vi "saved waveform analysis220915.vi"() -> ()   [LabVIEW 2024] (continued)
15774.841666666667, 15775.016666666666, 15774.108333333334, 15775.741666666667, 15777.991666666667, 15775.008333333333, 15781.708333333334, 15773.5, 15775.016666666666, 15770.058333333332, 15774.858333333334, 15789.625, 15781.283333333333, 15781.708333333334, 15784.266666666666, 15777.816666666668, 15776.033333333333, 15770.666666666666, 15776.8, 15864.675, 15911.983333333334, 15907.916666666666, 15908.383333333333, 15907.2, 15907.5, 15909.125, 15909.733333333334, 15911.133333333333, 15906.575, 15906.758333333333, 15910.95, 15902.566666666668, 15911.083333333334, 15905.275, 15902.716666666667, 15905.525, 15907.641666666666, 15912.85, 15907.9, 15907.341666666667, 15903.591666666667, 15905.575, 15913.883333333333, 15908.85, 15910.908333333333, 15908.683333333332, 15913.641666666666, 15901.641666666666, 15904.675, 15912.433333333332, 15909.3, 15912.441666666668, 15917.483333333334, 15911.675, 15913.625, 15908.708333333334, 15916.45, 15909.591666666667, 15907.508333333333, 15905.691666666668, 15913.183333333332, 15915.258333333333, 15907.341666666667, 15915.4, 15902.425, 15906.591666666667, 15910.916666666666, 15913.333333333334, 15917.041666666666, 15910.325, 15916.916666666666, 15912.408333333333, 15913.466666666667, 15916.125, 15916.783333333333, 15917.65, 15910.633333333333, 15915.608333333334, 15907.925, 15909.741666666667, 15907.925, 15911.05, 15913.466666666667, 15907.816666666668, 15906.0, 15916.591666666667, 15909.758333333333, 15912.575, 15907.8, 15912.283333333333, 15913.308333333332, 15906.741666666667, 15913.908333333333, 15909.133333333333, 15912.708333333334, 15908.391666666666, 15913.633333333333, 15914.216666666667, 15910.783333333333, 15906.758333333333, 15907.633333333333, 15909.866666666667, 15908.116666666667, 15917.383333333333, 15916.016666666666, 15911.983333333334, 15917.208333333334, 15912.716666666667, 15911.833333333334, 15901.35, 15913.141666666666, 15913.008333333333, 15913.625, 15914.241666666667, 15913.125, 15915.275, 15918.4, 15912.866666666667, 15910.183333333332, 15903.475, 15908.683333333332, 16035.166666666666, 16044.608333333334, 16048.633333333333, 16038.166666666666, 16052.491666666667, 16039.491666666667, 16038.008333333333, 16037.566666666668, 16042.833333333334, 16044.141666666666, 16042.95, 16041.766666666666, 16034.283333333333, 16042.641666666666, 16032.191666666668, 16036.658333333333, 16029.033333333333, 16030.383333333333, 16037.591666666667, 16044.733333333334, 16041.291666666666, 16037.866666666667, 16031.433333333332, 16038.633333333333, 16031.416666666666, 16044.133333333333, 16041.575, 16036.625, 16047.883333333333, 16035.483333333334, 16036.666666666666, 16033.1, 16037.558333333332, 16035.483333333334, 16030.541666666666, 16029.2, 16032.8, 16035.041666666666, 16037.425, 16035.333333333334, 16035.966666666667, 16035.758333333333, 16024.691666666668, 16035.175, 16034.766666666666, 16040.1, 16033.85, 16033.85, 16039.366666666667, 16037.416666666666, 16037.125, 16032.341666666667, 16027.091666666667, 16029.95, 16043.708333333334, 16038.008333333333, 16037.883333333333, 16034.716666666667, 16041.6, 16044.316666666668, 16035.933333333332, 16041.9, 16040.866666666667, 16041.208333333334, 16044.483333333334, 16037.408333333333, 16045.65, 16036.216666666667, 16040.733333333334, 16039.683333333332, 16042.491666666667, 16041.45, 16035.458333333334, 16042.841666666667, 16031.866666666667]]
  out "img scan":dbl[][](graph)
  out "sampling period [s]":dbl=2.0000000000000002e-07
  out "skip [us]":dbl=40.0
  out "element":dbl=5777979.0 format="%#.6g"
  in  "file path (use dialog)":path=path "F:/20220915-121218tdTomato-cropbulkcalib/waveforms.pico"
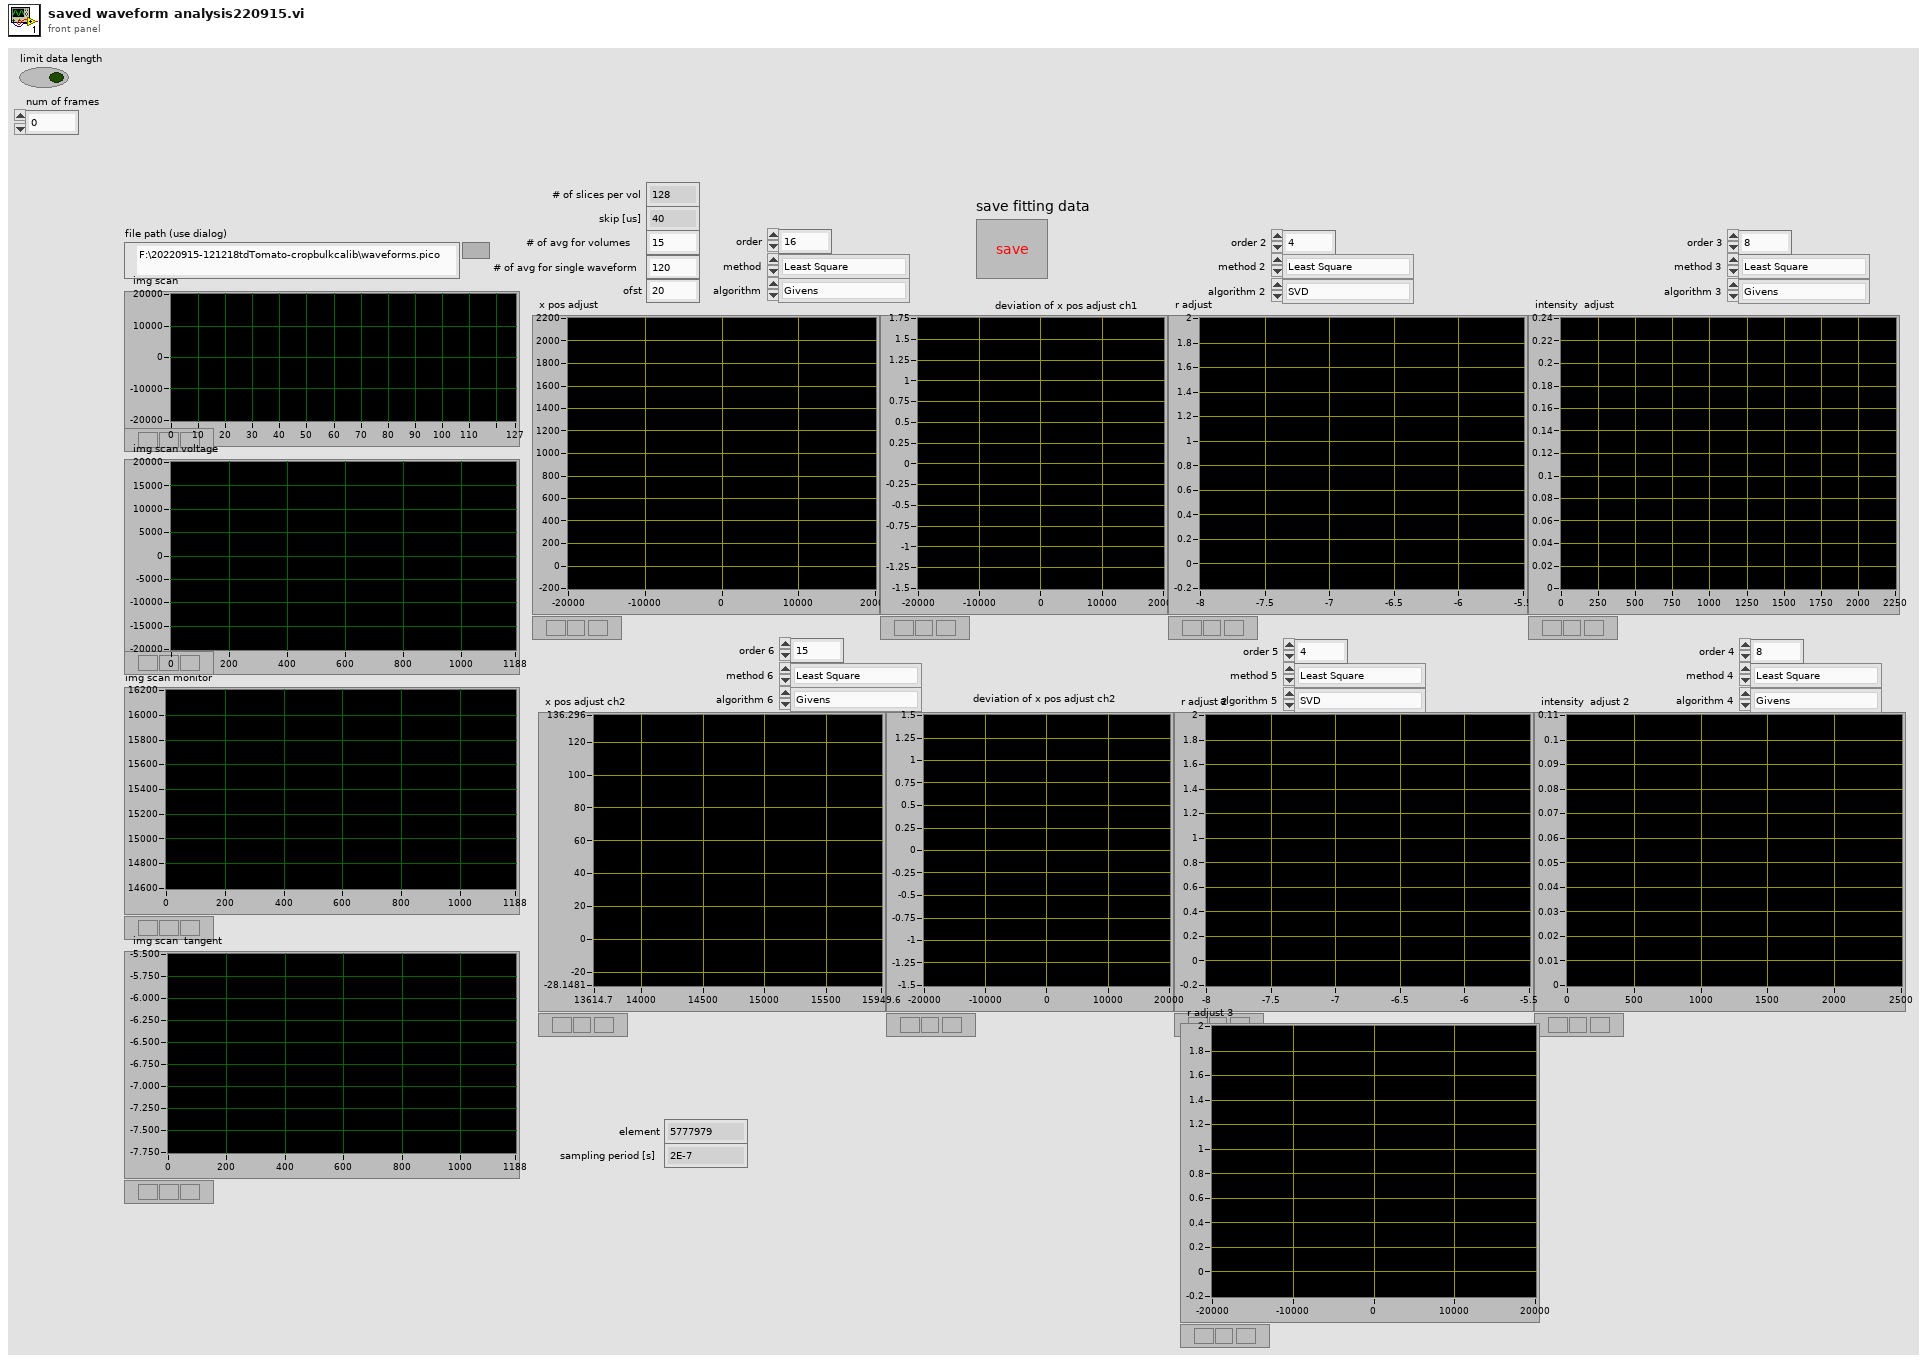
[diagram p1: front panel]
types:
  T1 = cluster{"img scan voltage":dbl[], "optimized param":dbl[]}
  T2 = cluster{"optimized param":dbl[], "Best Polynomial Fit":dbl[]}[]
  T3 = typedef "NI_AALPro.lvlib/Curve Fitting Criteria.ctl" = u16
  T4 = typedef "NI_AALPro.lvlib/General Linear Fit Algorithm.ctl" = u16
  T5 = cluster{"Array out":dbl[], "optimized param":dbl[]}[]
  T6 = cluster{"optimized param":dbl[], "optimized param":dbl[]}[]
  T7 = cluster{"# of avg for single waveform":u16, "skip [us]":dbl, "Nzf*Nv":i32, "ofst":dbl, "# of avg for volumes":u16, "limit data length":bool, "num of frames":i32, "Nv":i32}
  T8 = enum16{"open", "replace", "create", "open or create", "replace or create", "replace or create with confirmation"}
  T9 = cluster{"coeffs for r adjust":dbl[], "coeffs for x pos adjust":dbl[], "coeffs for intensity adjust":dbl[]}
  T10 = cluster{"config cluster":cluster{"xy cut pos correct":dbl[][], "3D reconst config":cluster{"xyz pos":u16[], "color 4":cluster{"color array":u32[], "num of colors":i32, "max":dbl, "min":dbl}, "autogain":bool, "zoom":dbl, "slice(T)/stack(F)":bool, "xy cut mag":dbl, "xy cut ofst":dbl, "z/xy comp":dbl, "y shift comp":dbl, "max plot":bool, "oblique angle [deg]":dbl, "voxel size z [um]":dbl, "voxel size xy[um]":dbl, "reverse v":bool, "reverse h":bool, "3D reconstruction":bool, "reverse z":bool}, "xy cut pos":dbl[][], "AOD scan speed ratio":dbl, "Nx":dbl, "stack method":enum16{"0pad to z", "0pad to x", "0pad to x and rot"}, "y shift":i32}, "optimized param":dbl[][][][][], "volume indices":i32[]}
  T11 = cluster{"img scan tangent":dbl[], "optimized param":dbl[]}
  T12 = cluster{"optimized param":dbl[], "optimized param":dbl[]}
  T13 = cluster{"img scan tangent":dbl[], "optimized param":dbl[]}[]
  T14 = cluster{"img scan voltage":dbl[], "optimized param":dbl[]}[]
  T15 = cluster{"coeffs for r adjust":dbl[], "coeffs for x pos adjust":dbl[], "coeffs for intensity adjust":dbl[]}[]
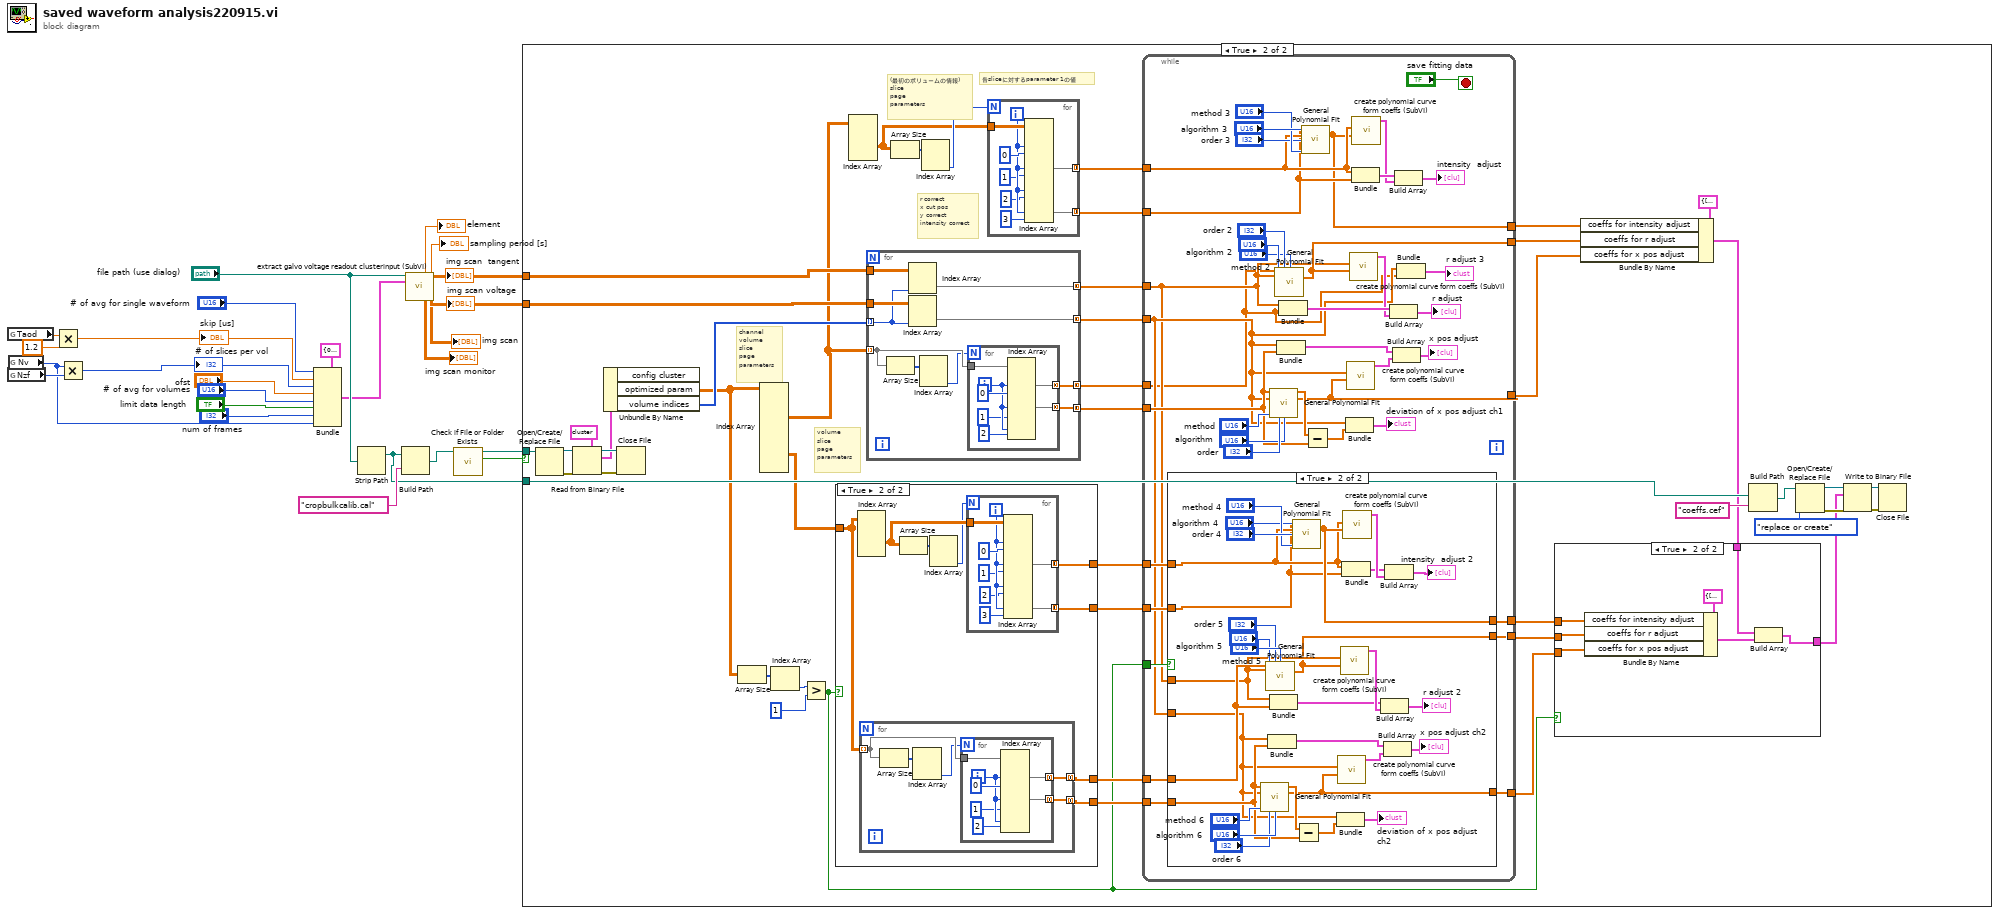
[diagram p0: block diagram]
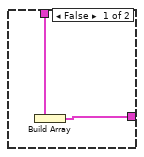
[diagram p3: hidden frame]
diagram:
  n1 = global read "global for picoscope.vi" "Taod"() -> (w13:dbl)
  n2 = global read "global for picoscope.vi" "Nzf"() -> (w11:i32)
  n3 = global read "global for picoscope.vi" "Nv"() -> (w2:i32)
  n4 = Multiply(x=w13, y=1.2) -> (x*y=w6:dbl)
  "skip [us]" <- w6
  n5 = Multiply(x=w2, y=w11) -> (x*y=w9:i32)
  "# of slices per vol" <- w9
  n6 = Bundle(cluster=T7 {"# of avg for single waveform"=0, "skip [us]"=0.0, "Nzf*Nv"=0, "ofst"=0.0, "# of avg for volumes"=0, "limit data length"=FALSE, "num of frames"=7500, "Nv"=8}, "# of avg for single waveform"="# of avg for single waveform", "skip [us]"=w6, "Nzf*Nv"=w9, "ofst"="ofst", "# of avg for volumes"="# of avg for volumes", "limit data length"="limit data length", "num of frames"="num of frames", "Nv"=w2) -> (w1:T7)
  n7 = Strip Path(path="file path (use dialog)") -> (stripped path=w18:path)  [unwired: 1 out]
  n8 = Build Path(base path=w18, name or relative path="cropbulkcalib.cal") -> (appended path=w20:path)
  n9 = call "extract galvo voltage readout clusterinput (SubVI).vi"("file path (use dialog)"="file path (use dialog)", "cluster"=w1) -> ("element"=→"element":dbl, "sampling period [s]"=→"sampling period [s]":dbl, "img scan tangent"=w24:dbl[][], "img scan voltage"=w23:dbl[][], "img scan monitor"=→"img scan monitor":dbl[][], "img scan"=→"img scan":dbl[][])  [unwired: 7 in, 1 out]
  "img scan voltage" <- w23
  "img scan  tangent" <- w24
  n10 = call <vilib>:"Check if File or Folder Exists.vi"("path"=w20) -> ("file or folder exists?"=w19:bool, "dup path"=w17:path)  [unwired: 8 in, 1 out]
  n11 = case shown="True" w19 {
    tunnel: w24 -> [_ w61]
    tunnel: w23 -> [_ w60]
    tunnel: w18 -> [_ w44]
    tunnel: w17 -> [_ w42]
    frame False {
    }
    frame True {
      # "r correct\nx cut pos\ny correct\nintensity correct"
      # "各sliceに対するparameter 1の値"
      # "(最初のボリュームの情報)\nslice\npage\nparameters"
      # "volume\nslice\npage\nparameters"
      # "channel\nvolume\nslice\npage\nparameters"
      n12 = Open/Create/Replace File(file path (use dialog)=w42) -> (refnum out=w71:refnum<file>, error out=w70:errorcluster)  [unwired: 5 in, 1 out]
      n13 = Read from Binary File(5:T10 {"config cluster"={"xy cut pos correct"=[], "3D reconst config"={"xyz pos"=[], "color 4"={"color array"=[], "num of colors"=0, "max"=0.0, "min"=0.0}, "autogain"=FALSE, "zoom"=0.0, "slice(T)/stack(F)"=FALSE, "xy cut mag"=0.0, "xy cut ofst"=0.0, "z/xy comp"=0.0, "y shift comp"=0.0, "max plot"=FALSE, "oblique angle [deg]"=0.0, "voxel size z [um]"=0.0, "voxel size xy[um]"=0.0, "reverse v"=FALSE, "reverse h"=FALSE, "3D reconstruction"=FALSE, "reverse z"=FALSE}, "xy cut pos"=[], "AOD scan speed ratio"=0.0, "Nx"=0.0, "stack method"=enum."0pad to z", "y shift"=0}, "optimized param"=[], "volume indices"=[]} ("cluster"), 8:w70, 11:w71) -> (0:w69:errorcluster, 2:w67:T10, 3:w68:refnum<file>)  [unwired: 3 in, 1 out]
      n14 = Unbundle By Name(w67) -> ("optimized param"=w35:dbl[][][][][], "volume indices"=w66:i32[])  [unwired: 1 out]
      n15 = Close File(refnum=w68, error in=w69) -> ()  [unwired: 2 out]
      n16 = Array Size(array=w35) -> (size(s)=w34:i32[])
      n17 = Index Array(array=w35) -> (element #1=w55:dbl[][][][], element #2=w40:dbl[][][][])  [unwired: 10 in]
      n18 = Index Array(array=w34) -> (element=w33:i32)  [unwired: 1 in]
      n19 = Greater?(x=w33, y=1) -> (0:w26:bool)
      n20 = case shown="True" w26 {
        tunnel: w40 -> [_ w86]
        tunnel: [_ w85] -> w39
        tunnel: [_ w84] -> w38
        tunnel: [_ w83] -> w37
        tunnel: [_ w82] -> w36
        frame False {
        }
        frame True {
          n21 = Index Array(array=w86) -> (element=w89:dbl[][][])  [unwired: 4 in]
          n22 = for {
            tunnel: w86 -> [w93] mode=indexing
            tunnel: [w91] -> w84 mode=concatenating
            tunnel: [w90] -> w85 mode=concatenating
            n23 = Array Size(array=w93) -> (size(s)=w94:i32[])
            n24 = Index Array(array=w94) -> (element #2=w92:i32)  [unwired: 2 in, 1 out]
            n25 = for {
              N: w92 -> [_]
              tunnel: w93 -> [w101]
              tunnel: [w96] -> w91 mode=concatenating
              tunnel: [w95] -> w90 mode=concatenating
              i -> [w99]
              n26 = Index Array(array=w101, index (dim 1) #1=w99, index (dim 2) #1=0 ("disabled index (col)"), index (dim 1) #2=w99, index (dim 2) #2=1 ("disabled index (col)"), index (dim 1) #3=w99, index (dim 2) #3=2 ("disabled index (col)")) -> (element #1=w95:dbl[], element #2=w96:dbl[])  [unwired: 3 in, 1 out]
            }
          }
          n27 = Array Size(array=w89) -> (size(s)=w88:i32[])
          n28 = Index Array(array=w88) -> (element #2=w87:i32)  [unwired: 2 in, 1 out]
          n29 = for {
            N: w87 -> [_]
            tunnel: w89 -> [w109]
            tunnel: [w103] -> w83 mode=concatenating
            tunnel: [w102] -> w82 mode=concatenating
            i -> [w107]
            n30 = Index Array(array=w109, index (dim 1) #1=w107, index (dim 2) #1=0 ("disabled index (col)"), index (dim 1) #2=w107, index (dim 2) #2=1 ("disabled index (col)"), index (dim 1) #3=w107, index (dim 2) #3=2 ("disabled index (col)"), index (dim 1) #4=w107, index (dim 2) #4=3 ("disabled index (col)")) -> (element #2=w103:dbl[], element #4=w102:dbl[])  [unwired: 4 in, 2 out]
          }
        }
      }
      n31 = Index Array(array=w55) -> (element=w54:dbl[][][])  [unwired: 4 in]
      n32 = for {
        tunnel: w66 -> [w190] mode=indexing
        tunnel: w55 -> [w195] mode=indexing
        tunnel: w60 -> [w197]
        tunnel: [w193] -> w65 mode=concatenating
        tunnel: [w192] -> w64 mode=concatenating
        tunnel: [w191] -> w63 mode=concatenating
        tunnel: w61 -> [w189]
        tunnel: [w188] -> w62 mode=concatenating
        n33 = Array Size(array=w195) -> (size(s)=w196:i32[])
        n34 = Index Array(array=w189, index (col)=w190) -> (element=w188:dbl[])  [unwired: 1 in]
        n35 = Index Array(array=w197, index (col)=w190) -> (element=w193:dbl[])  [unwired: 1 in]
        n36 = Index Array(array=w196) -> (element #2=w194:i32)  [unwired: 2 in, 1 out]
        n37 = for {
          N: w194 -> [_]
          tunnel: w195 -> [w204]
          tunnel: [w199] -> w192 mode=concatenating
          tunnel: [w198] -> w191 mode=concatenating
          i -> [w202]
          n38 = Index Array(array=w204, index (dim 1) #1=w202, index (dim 2) #1=0 ("disabled index (col)"), index (dim 1) #2=w202, index (dim 2) #2=1 ("disabled index (col)"), index (dim 1) #3=w202, index (dim 2) #3=2 ("disabled index (col)")) -> (element #1=w198:dbl[], element #2=w199:dbl[])  [unwired: 3 in, 1 out]
        }
      }
      n39 = Array Size(array=w54) -> (size(s)=w58:i32[])
      n40 = Index Array(array=w58) -> (element #2=w59:i32)  [unwired: 2 in, 1 out]
      n41 = for {
        N: w59 -> [_]
        tunnel: w54 -> [w117]
        tunnel: [w111] -> w56 mode=concatenating
        tunnel: [w110] -> w57 mode=concatenating
        i -> [w115]
        n42 = Index Array(array=w117, index (dim 1) #1=w115, index (dim 2) #1=0 ("disabled index (col)"), index (dim 1) #2=w115, index (dim 2) #2=1 ("disabled index (col)"), index (dim 1) #3=w115, index (dim 2) #3=2 ("disabled index (col)"), index (dim 1) #4=w115, index (dim 2) #4=3 ("disabled index (col)")) -> (element #2=w111:dbl[], element #4=w110:dbl[])  [unwired: 4 in, 2 out]
      }
      n43 = while {
        tunnel: w65 -> [w120]
        tunnel: w64 -> [w142]
        tunnel: w63 -> [w118]
        tunnel: w62 -> [w119]
        tunnel: w57 -> [w136]
        tunnel: w56 -> [w137]
        tunnel: [w133] -> w53
        tunnel: [w132] -> w52
        tunnel: [w130] -> w51
        tunnel: w39 -> [w129]
        tunnel: w38 -> [w128]
        tunnel: [w127] -> w31
        tunnel: [w126] -> w30
        tunnel: [w125] -> w29
        tunnel: w37 -> [w124]
        tunnel: w36 -> [w123]
        tunnel: w26 -> [w122]
        stop <- "save fitting data" stop-if-true
        n44 = case shown="True" w122 {
          tunnel: w129 -> [_ w166]
          tunnel: w128 -> [_ w165]
          tunnel: w119 -> [_ w164]
          tunnel: w120 -> [_ w163]
          tunnel: [_ w162] -> w127
          tunnel: [_ w161] -> w126
          tunnel: [_ w160] -> w125
          tunnel: w124 -> [_ w159]
          tunnel: w123 -> [_ w158]
          frame False {
          }
          frame True {
            n45 = call <vilib>:"General Polynomial Fit.vi"("Y"=w165, "polynomial order"="order 6", "X"=w163, "method"="method 6", "algorithm"="algorithm 6") -> ("Best Polynomial Fit"=w187:dbl[], "Polynomial Coefficients"=w160:dbl[])  [unwired: 7 in, 2 out]
            n46 = call <vilib>:"General Polynomial Fit.vi"("Y"=w166, "polynomial order"="order 5", "X"=w164, "method"="method 5", "algorithm"="algorithm 5") -> ("Polynomial Coefficients"=w161:dbl[])  [unwired: 7 in, 3 out]
            n47 = Bundle("img scan voltage"=w163, "optimized param"=w165) -> (w167:T1)  [unwired: 1 in]
            n48 = Bundle("img scan tangent"=w164, "optimized param"=w166) -> (w178:T11)  [unwired: 1 in]
            n49 = call <vilib>:"General Polynomial Fit.vi"("Y"=w158, "polynomial order"="order 4", "X"=w159, "method"="method 4", "algorithm"="algorithm 4") -> ("Polynomial Coefficients"=w162:dbl[])  [unwired: 7 in, 3 out]
            n50 = Subtract(x=w187, y=w165) -> (x-y=w169:dbl[])
            n51 = Bundle("img scan voltage"=w163, w169) -> (→"deviation of x pos adjust ch2":cluster{"img scan voltage":dbl[], dbl[]})  [unwired: 1 in]
            n52 = call "create polynomial curve form coeffs (SubVI).vi"("Polynomial Coefficients"=w160, "input data"=w163) -> ("Cluster"=w174:cluster{dbl[], dbl[]})  [unwired: 9 in]
            n53 = call "create polynomial curve form coeffs (SubVI).vi"("Polynomial Coefficients"=w161, "input data"=w164) -> ("Cluster"=w179:cluster{dbl[], dbl[]})  [unwired: 9 in]
            n54 = Bundle("optimized param"=w159, "optimized param"=w158) -> (w185:T12)  [unwired: 1 in]
            n55 = call "create polynomial curve form coeffs (SubVI).vi"("Polynomial Coefficients"=w162, "input data"=w159) -> ("Cluster"=w186:cluster{dbl[], dbl[]})  [unwired: 9 in]
            n56 = Build Array(w178, w179) -> (→"r adjust 2":T13)
            n57 = Build Array(w167, w174) -> (→"x pos adjust ch2":T14)
            n58 = Build Array(w185, w186) -> (→"intensity  adjust 2":T6)
          }
        }
        n59 = call <vilib>:"General Polynomial Fit.vi"("Y"=w142, "polynomial order"="order", "X"=w120, "method"="method", "algorithm"="algorithm") -> ("Best Polynomial Fit"=w131:dbl[], "Polynomial Coefficients"=w130:dbl[])  [unwired: 7 in, 2 out]
        n60 = call <vilib>:"General Polynomial Fit.vi"("Y"=w118, "polynomial order"="order 2", "X"=w119, "method"="method 2", "algorithm"="algorithm 2") -> ("Polynomial Coefficients"=w132:dbl[])  [unwired: 7 in, 3 out]
        n61 = Bundle("img scan voltage"=w120, "optimized param"=w142) -> (w157:T1)  [unwired: 1 in]
        n62 = Bundle("img scan tangent"=w119, "optimized param"=w118) -> (w145:T11)  [unwired: 1 in]
        n63 = call <vilib>:"General Polynomial Fit.vi"("Y"=w136, "polynomial order"="order 3", "X"=w137, "method"="method 3", "algorithm"="algorithm 3") -> ("Polynomial Coefficients"=w133:dbl[])  [unwired: 7 in, 3 out]
        n64 = Subtract(x=w131, y=w142) -> (x-y=w155:dbl[])
        n65 = Bundle("img scan voltage"=w120, w155) -> (→"deviation of x pos adjust ch1":cluster{"img scan voltage":dbl[], dbl[]})  [unwired: 1 in]
        n66 = call "create polynomial curve form coeffs (SubVI).vi"("Polynomial Coefficients"=w130, "input data"=w120) -> ("Cluster"=w149:cluster{dbl[], dbl[]})  [unwired: 9 in]
        n67 = call "create polynomial curve form coeffs (SubVI).vi"("Polynomial Coefficients"=w132, "input data"=w119) -> ("Cluster"=w144:cluster{dbl[], dbl[]})  [unwired: 9 in]
        n68 = Bundle("optimized param"=w137, "optimized param"=w136) -> (w135:T12)  [unwired: 1 in]
        n69 = call "create polynomial curve form coeffs (SubVI).vi"("Polynomial Coefficients"=w133, "input data"=w137) -> ("Cluster"=w134:cluster{dbl[], dbl[]})  [unwired: 9 in]
        n70 = Build Array(w145, w144) -> (→"r adjust":T13)
        n71 = Build Array(w157, w149) -> (→"x pos adjust":T14)
        n72 = Build Array(w135, w134) -> (→"intensity  adjust":T6)
        n73 = Bundle("img scan voltage"=w120, "optimized param"=w118) -> (→"r adjust 3":T1)  [unwired: 1 in]
      }
      n74 = Bundle By Name(cluster=T9 {"coeffs for r adjust"=[], "coeffs for x pos adjust"=[], "coeffs for intensity adjust"=[]}, "coeffs for intensity adjust"=w53, "coeffs for r adjust"=w52, "coeffs for x pos adjust"=w51) -> (w28:T9)
      n75 = case shown="True" w26 {
        tunnel: w31 -> [_ w80]
        tunnel: w30 -> [_ w79]
        tunnel: w29 -> [_ w78]
        tunnel: w28 -> [w74 w77]
        tunnel: [w73 w75] -> w27
        frame False {
          n76 = Build Array(w74) -> (w73:T15)
        }
        frame True {
          n77 = Bundle By Name(cluster=T9 {"coeffs for r adjust"=[], "coeffs for x pos adjust"=[], "coeffs for intensity adjust"=[]}, "coeffs for intensity adjust"=w80, "coeffs for r adjust"=w79, "coeffs for x pos adjust"=w78) -> (w76:T9)
          n78 = Build Array(w77, w76) -> (w75:T15)
        }
      }
      n79 = Build Path(base path=w44, name or relative path="coeffs.cef") -> (appended path=w45:path)
      n80 = Open/Create/Replace File(file path (use dialog)=w45, operation (0:open)=T8."replace or create") -> (refnum out=w46:refnum<file>, error out=w47:errorcluster)  [unwired: 4 in, 1 out]
      n81 = Write to Binary File(file (use dialog)=w46, data=w27, error in=w47) -> (refnum out=w49:refnum<file>, error out=w48:errorcluster)  [unwired: 3 in, 1 out]
      n82 = Close File(refnum=w49, error in=w48) -> ()  [unwired: 2 out]
    }
  }
